vi "flyVideoAcquisition.vi"(6 "image format controls":T1={"Pixel Format"="YUV 422 Packed", "width"=2448, "height"=900, "sub image height"=600, "sub image width"=1200}, 7 "image selector":u16(ring) items=["raw image", "single channel", "focus check", "downsampled", "subtraction result", "thresholded", "filtered", "cleaned", "cropped"], 8 "resave BG time":u32=10, 9 "image cluster":T4={"raw"="raw", "single channel"="single channel", "focus check"="focus check", "downsampled"="downsampled", "subtraction"="subtraction", "thresholded"="thresholded", "filtered"="filtered", "cleaned"="cleaned", "cropped"="cropped"}, 10 "im proc controls":T5={"Color Plane"=2, "downsampling"=32, "Filter"=enum."AutoM", "Number of Erosions"=2, "Focus threshold"=20.0, "Focus std threshold"=0.0, "background\nsubtraction"=TRUE, "Threshold"=121} {"Threshold" scale=0.0..255.0; "Color Plane" items=["Red", "Green", "Blue", "Hue", "Saturation", "Luminance", "Value", "Intensity"]}, 11 "status":T2(ring)=enum."fly in chamber") -> (0 "image out":T3, 1 "processed FPS":dbl=20.114942528735632, 2 "acquired FPS":dbl=20.114942528735632, 3 "acquiring video":bool)   [LabVIEW 2012]
uses:
  <vilib>/vision/Image Controls.llb/IMAQ Image.ctl
  GlobalBaslerCamera.vi
panel:
  out "Buffer Number Out":u32=984
  out "Number of Particles":i32
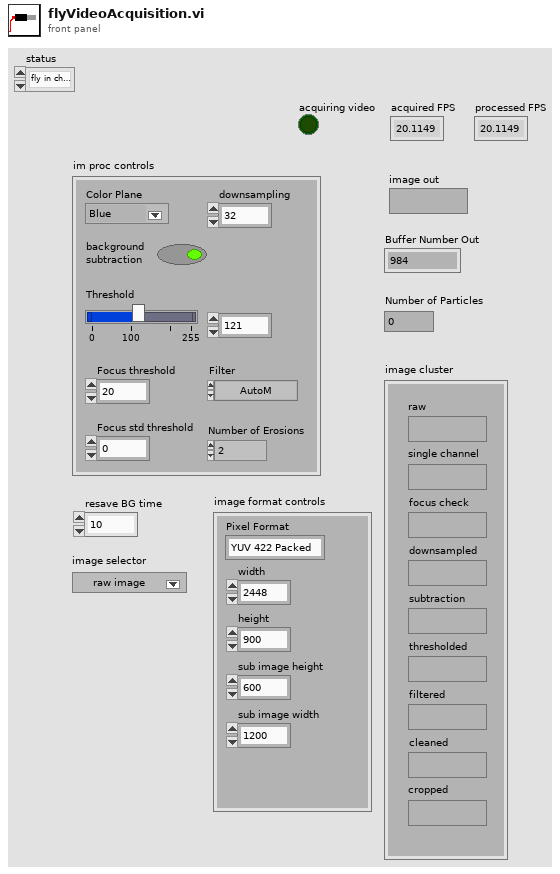
[diagram p1: front panel]
types:
  T1 = cluster{"Pixel Format":string, "width":u32, "height":u32, "sub image height":u32, "sub image width":u32}
  T2 = enum16{"waiting for fly", "closing gate", "fly in chamber", "taking decision", "keeping the fly", "blowing back", "activate flies"}
  T3 = typedef "IMAQ Image.ctl" = refnum<image>
  T4 = cluster{"raw":T3, "single channel":T3, "focus check":T3, "downsampled":T3, "subtraction":T3, "thresholded":T3, "filtered":T3, "cleaned":T3, "cropped":T3}
  T5 = cluster{"Color Plane":i32, "downsampling":i32, "Filter":enum32{"AutoM", "Close", "Dilate", "Erode", "Gradient", "Gradient out", "Gradient in", "Hit miss", "Open", "PClose", "POpen", "Thick", "Thin"}, "Number of Erosions":i32, "Focus threshold":sgl, "Focus std threshold":sgl, "background\nsubtraction":bool, "Threshold":u8}
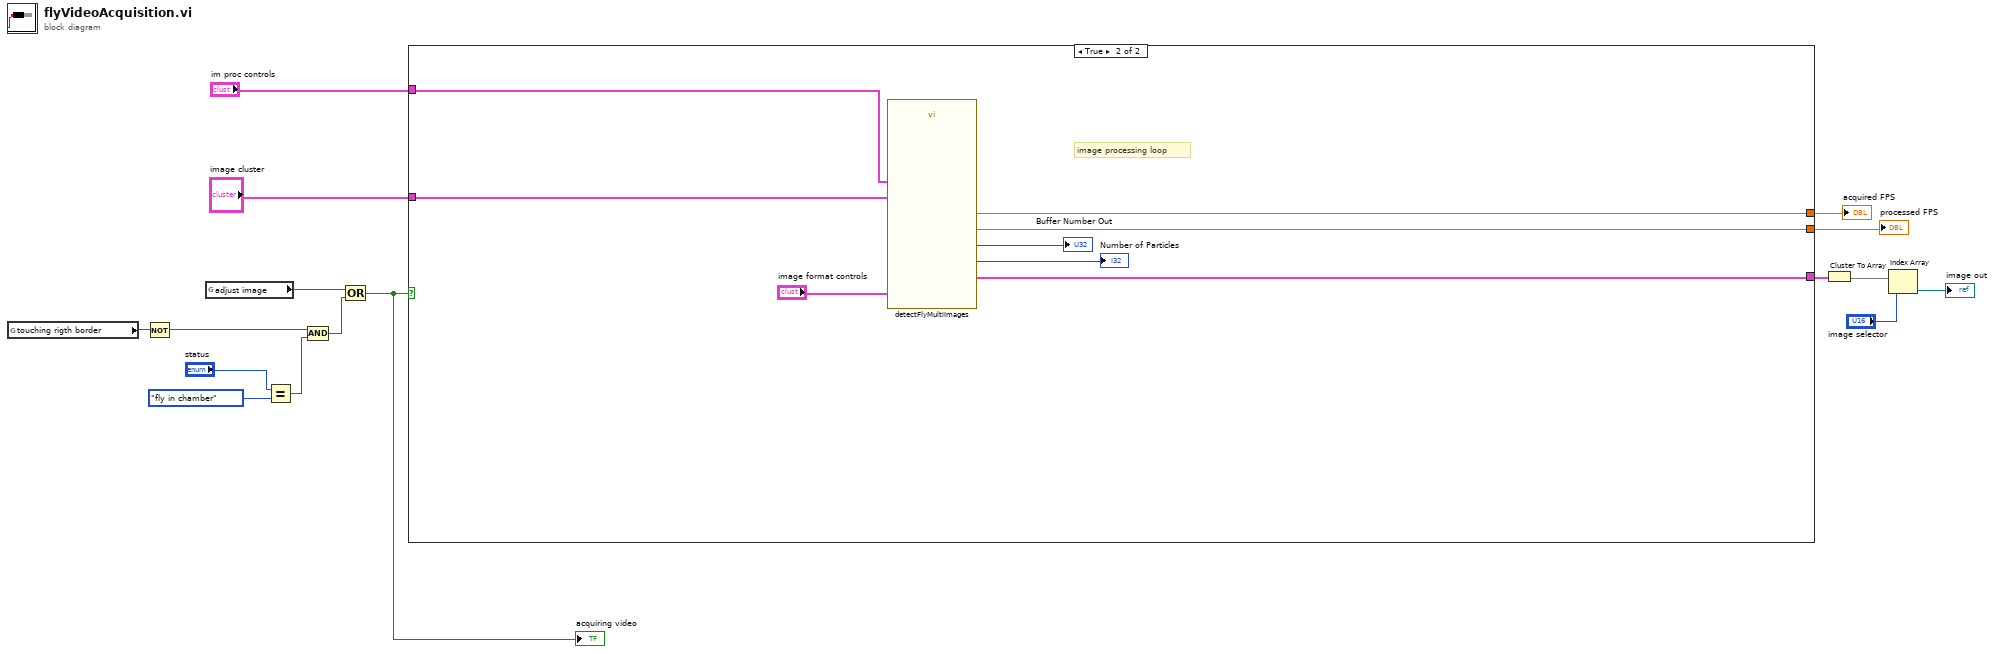
[diagram p0: block diagram]
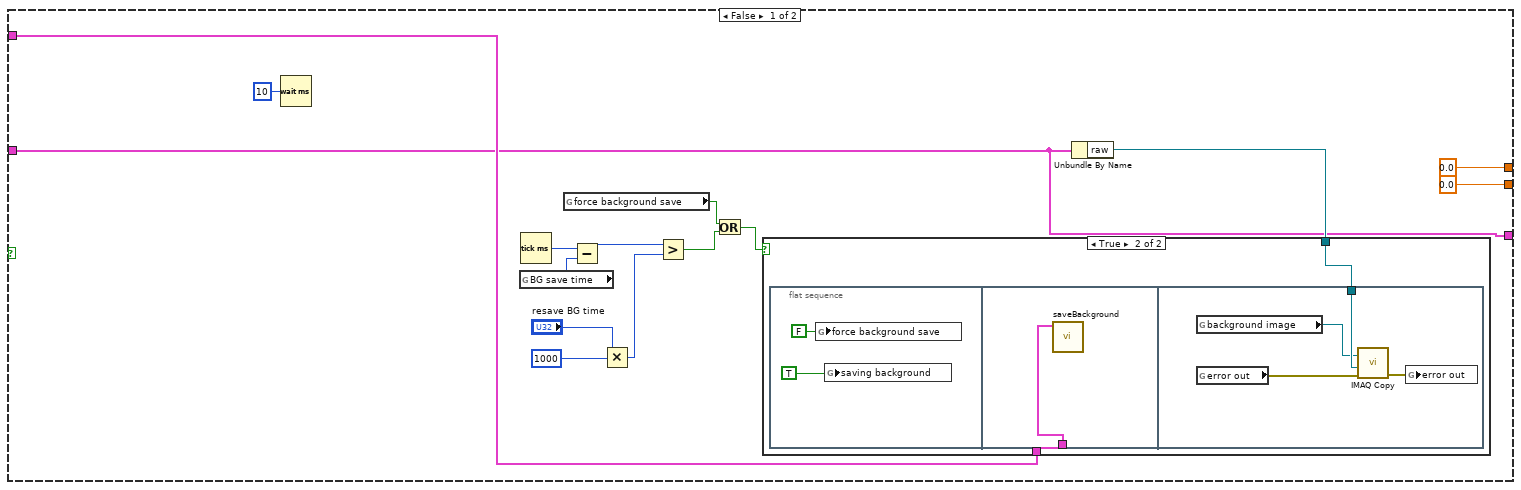
[diagram p2: hidden frame]
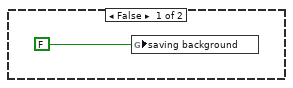
[diagram p3: hidden frame]
diagram:
  n1 = global read "GlobalBaslerCamera.vi" "touching rigth border"() -> (w4:bool)
  n2 = Not(x=w4) -> (.not. x?=w3:bool)
  n3 = global read "GlobalBaslerCamera.vi" "adjust image"() -> (w8:bool)
  n4 = Equal?(x="status", y=T2."fly in chamber") -> (x = y?=w6:bool)
  n5 = And(x=w3, y=w6) -> (x .and. y?=w7:bool)
  n6 = Or(x=w8, y=w7) -> (x .or. y?=w5:bool)
  "acquiring video" <- w5
  n7 = case shown="True" w5 {
    tunnel: [0.0 ("processed FPS") w44] -> w16
    tunnel: [0.0 ("acquired FPS") w45] -> w15
    tunnel: "im proc controls" -> [w23 w47]
    tunnel: "image cluster" -> [w21 w46]
    tunnel: [w21 w43] -> w10
    frame False {
      n8 = Wait (ms)(milliseconds to wait=u32 10) -> ()  [unwired: 1 out]
      n9 = global read "GlobalBaslerCamera.vi" "BG save time"() -> (w31:i64)
      n10 = Tick Count (ms)() -> (millisecond timer value=w24:u32)
      n11 = global read "GlobalBaslerCamera.vi" "force background save"() -> (w19:bool)
      n12 = Subtract(x=w24, y=w31) -> (x-y=w28:i64)
      n13 = Multiply(x="resave BG time", y=u32 1000) -> (x*y=w27:u32)
      n14 = Greater?(x=w28, y=w27) -> (0:w18:bool)
      n15 = Or(x=w19, y=w18) -> (x .or. y?=w17:bool)
      n16 = Unbundle By Name(w21) -> ("raw"=w22:T3)
      n17 = case shown="True" w17 {
        tunnel: w23 -> [_ w34]
        tunnel: w22 -> [_ w33]
        frame False {
          n18 = global write "GlobalBaslerCamera.vi" "saving background"(FALSE) -> ()
        }
        frame True {
          n19 = flat-sequence {
            tunnel: w34 -> [w37]
            tunnel: w33 -> [w39]
            frame #0 {
              n20 = global write "GlobalBaslerCamera.vi" "force background save"(FALSE ("force background save")) -> ()
              n21 = global write "GlobalBaslerCamera.vi" "saving background"(TRUE) -> ()
            }
            frame #1 {
              n22 = call "saveBackground.vi"("im proc controls"=w37) -> ()  [unwired: 11 in]
            }
            frame #2 {
              n23 = global read "GlobalBaslerCamera.vi" "background image"() -> (w38:T3)
              n24 = global read "GlobalBaslerCamera.vi" "error out"() -> (w41:errorcluster)
              n25 = call "IMAQ Copy"("error in (no error)"=w41, "Image Dst"=w39, "Image Src"=w38) -> ("error out"=w40:errorcluster)  [unwired: 3 in, 1 out]
              n26 = global write "GlobalBaslerCamera.vi" "error out"(w40) -> ()
            }
          }
        }
      }
    }
    frame True {
      # "image processing loop"
      n27 = call "detectFlyMultiImages.vi"("im proc controls"=w47, "image cluster"=w46, "image format controls"="image format controls") -> ("acquired FPS"=w45:dbl, "processed FPS"=w44:dbl, "Number of Particles"=→"Number of Particles":i32, "Buffer Number Out"=→"Buffer Number Out":u32, "image cluster out"=w43:T4)  [unwired: 8 in]
    }
  }
  "processed FPS" <- w16
  "acquired FPS" <- w15
  n28 = Cluster To Array(cluster=w10) -> (array=w11:T3[])
  n29 = Index Array(array=w11, index="image selector") -> (element=→"image out":T3)
